vi "CRYO_MASTER_FULL_IP.vi"() -> ()   [LabVIEW 2017] (continued)
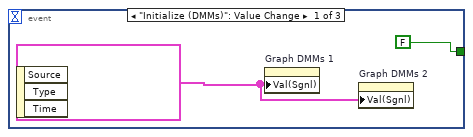
[diagram p2: hidden frame]
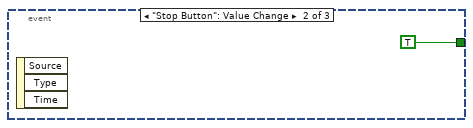
[diagram p3: hidden frame]
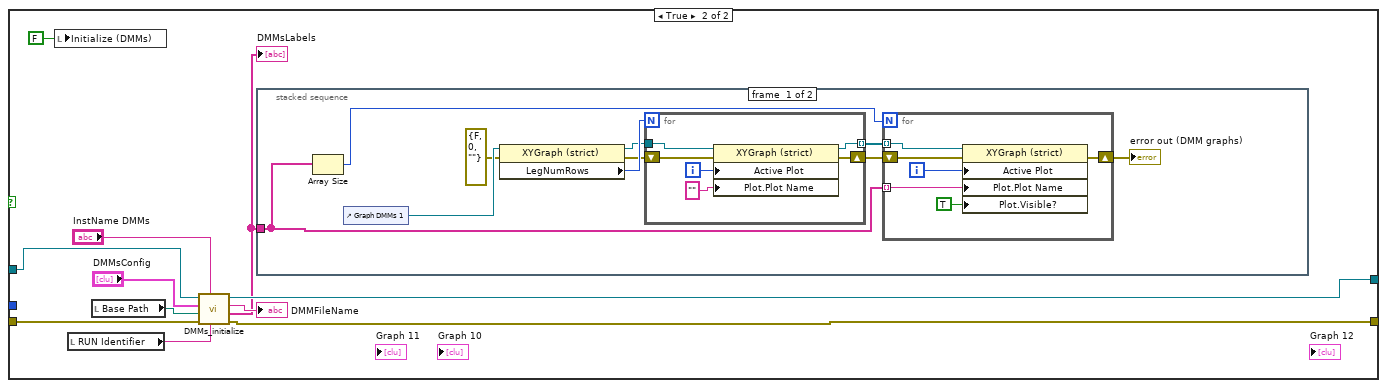
[diagram p5: hidden frame]
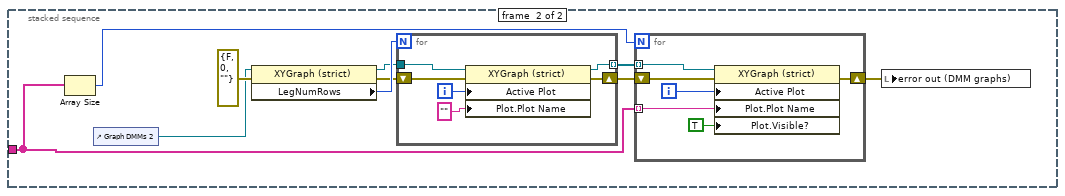
[diagram p6: hidden frame]
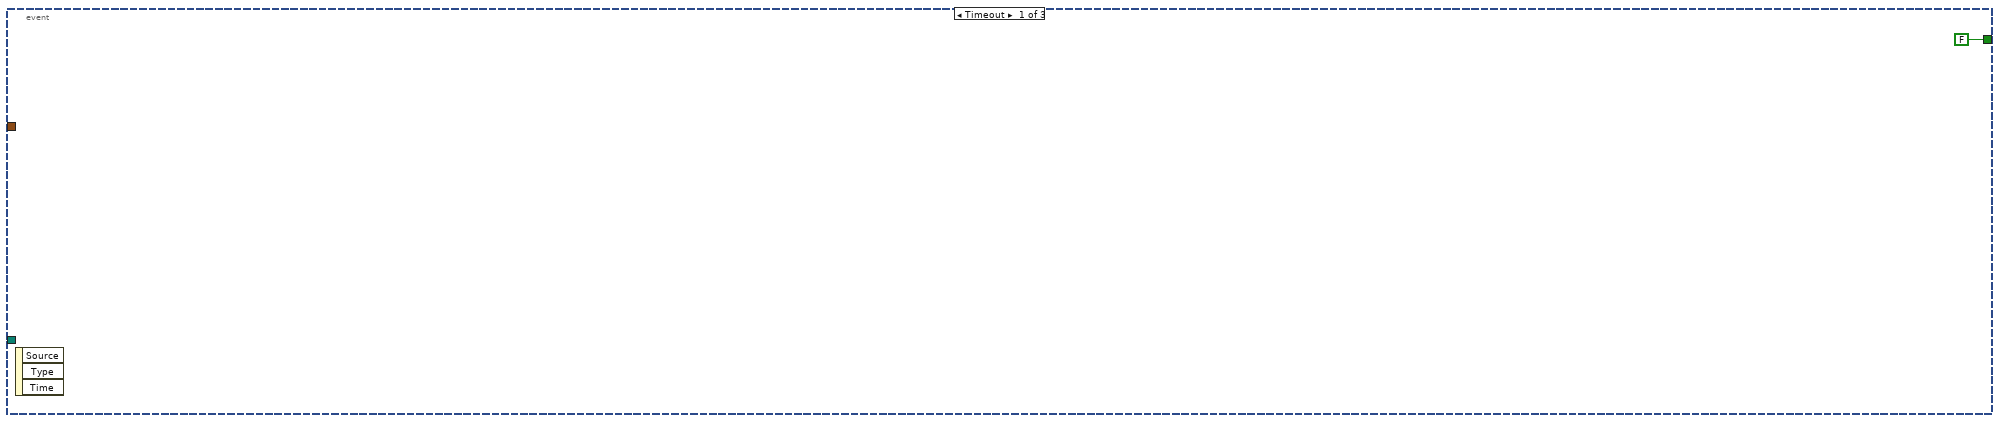
[diagram p7: hidden frame]
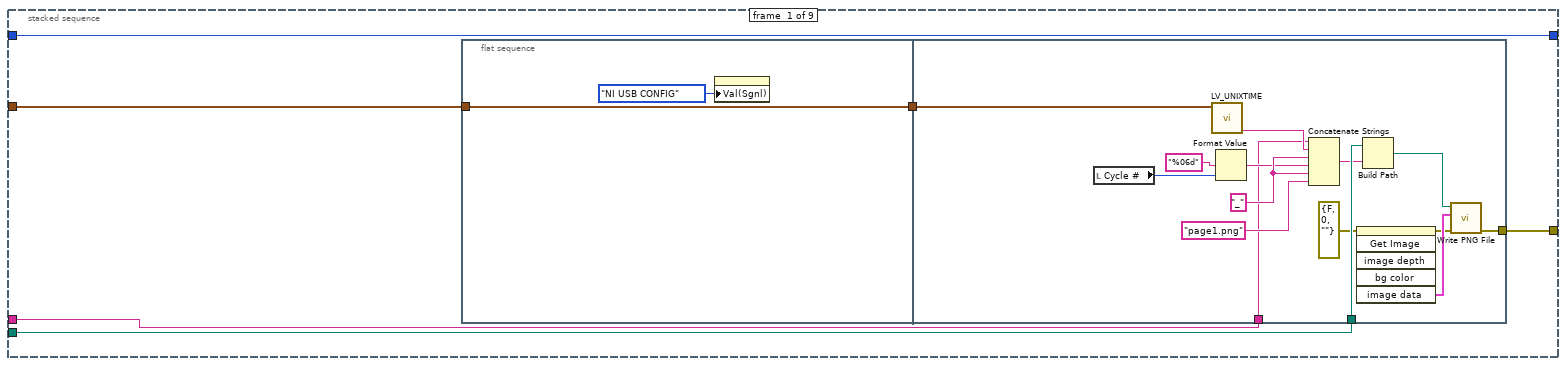
[diagram p8: hidden frame]
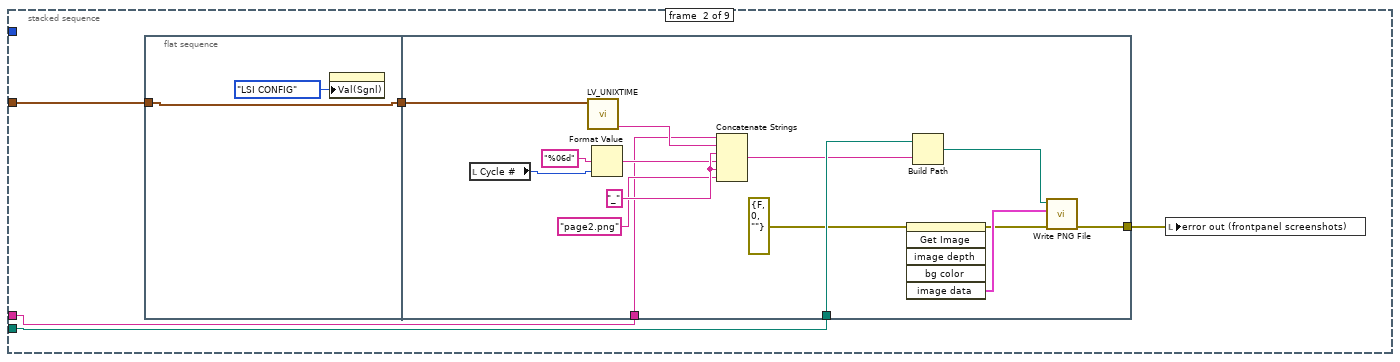
[diagram p9: hidden frame]
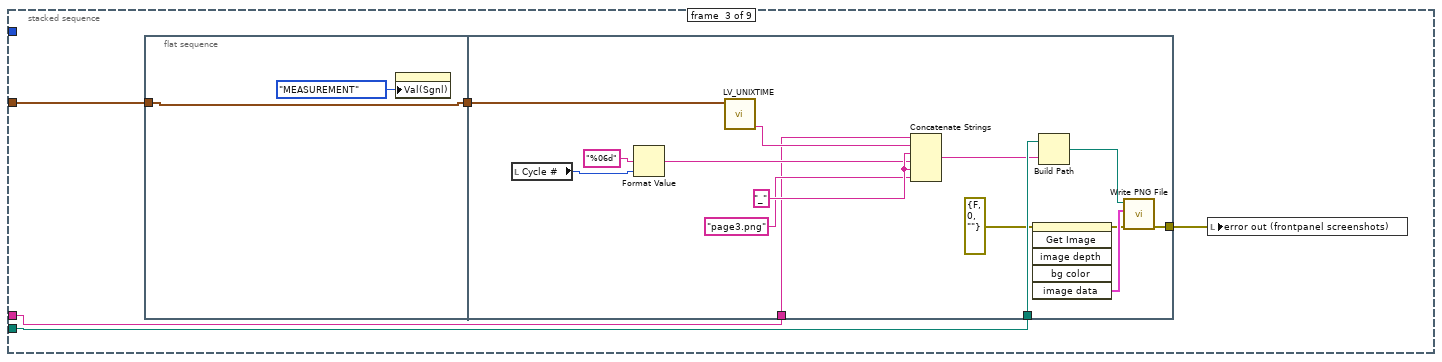
[diagram p10: hidden frame]
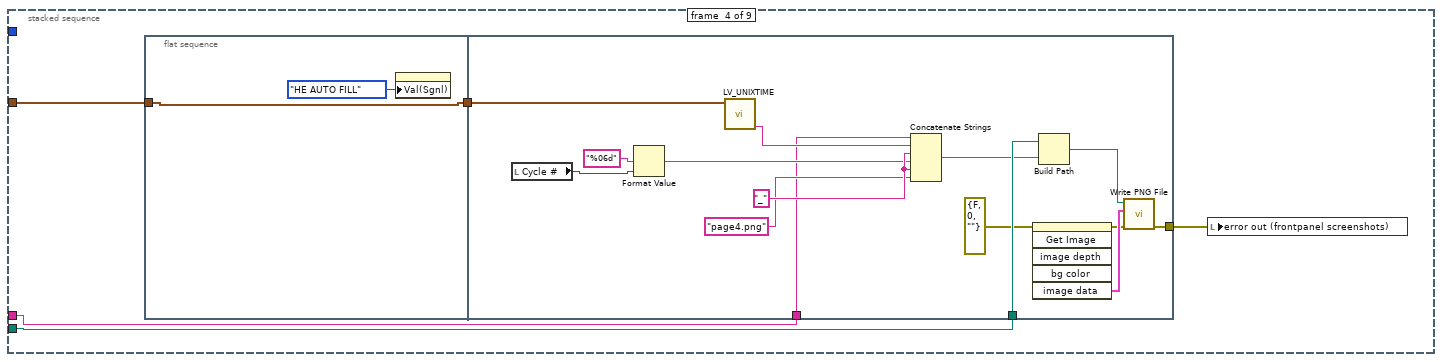
[diagram p11: hidden frame]
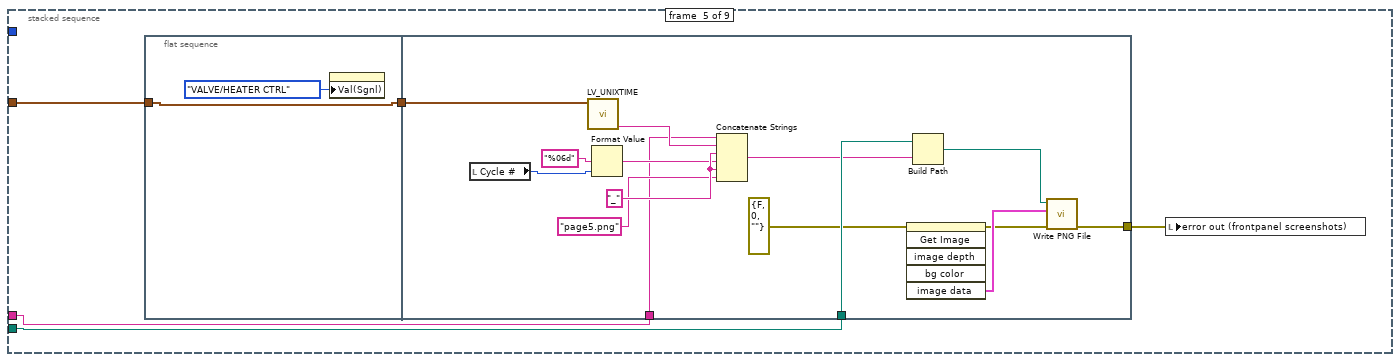
[diagram p12: hidden frame]
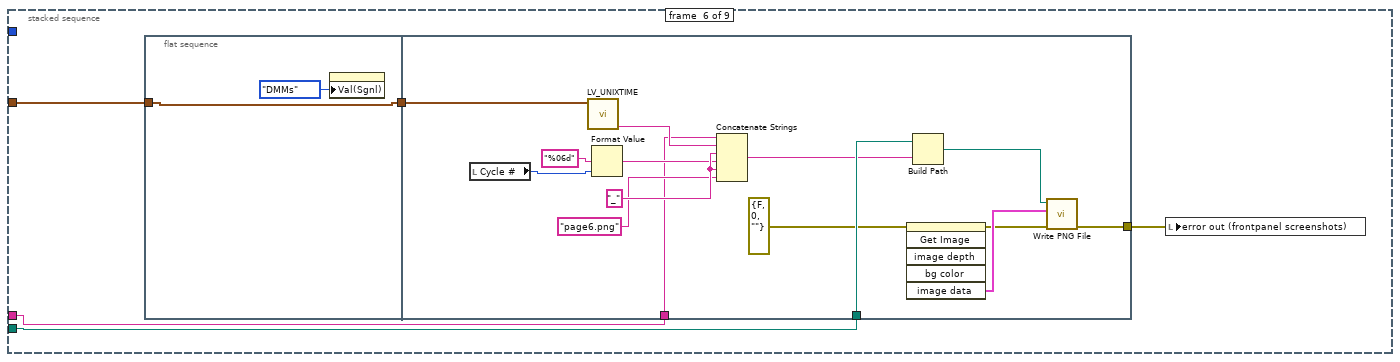
[diagram p13: hidden frame]
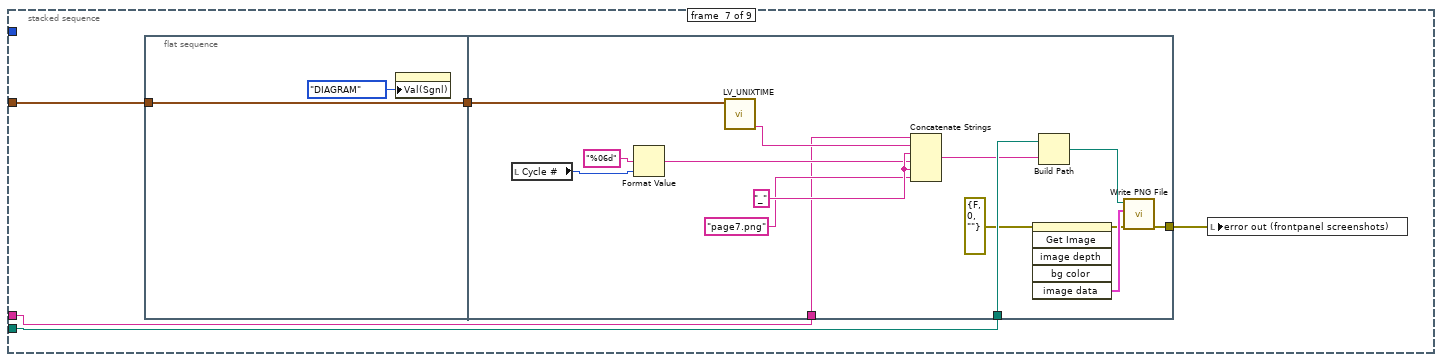
[diagram p14: hidden frame]
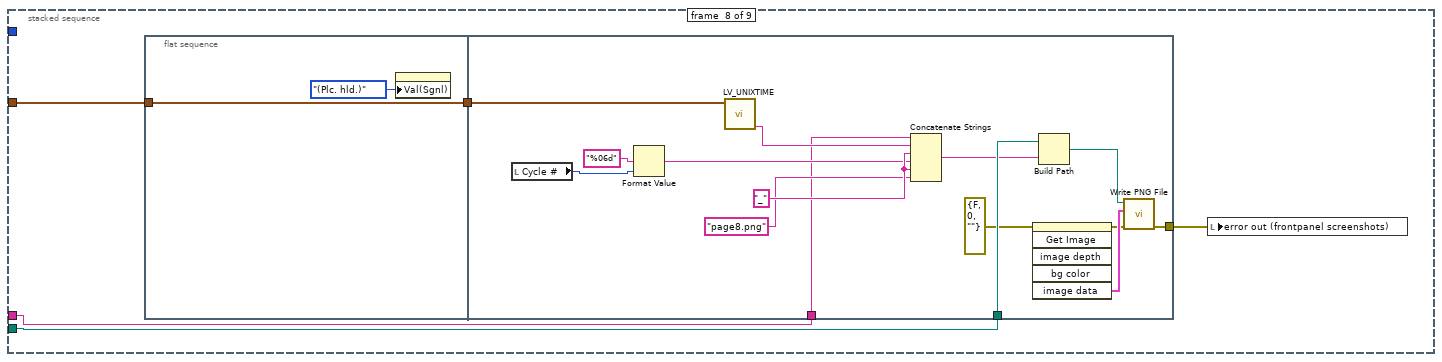
[diagram p15: hidden frame]
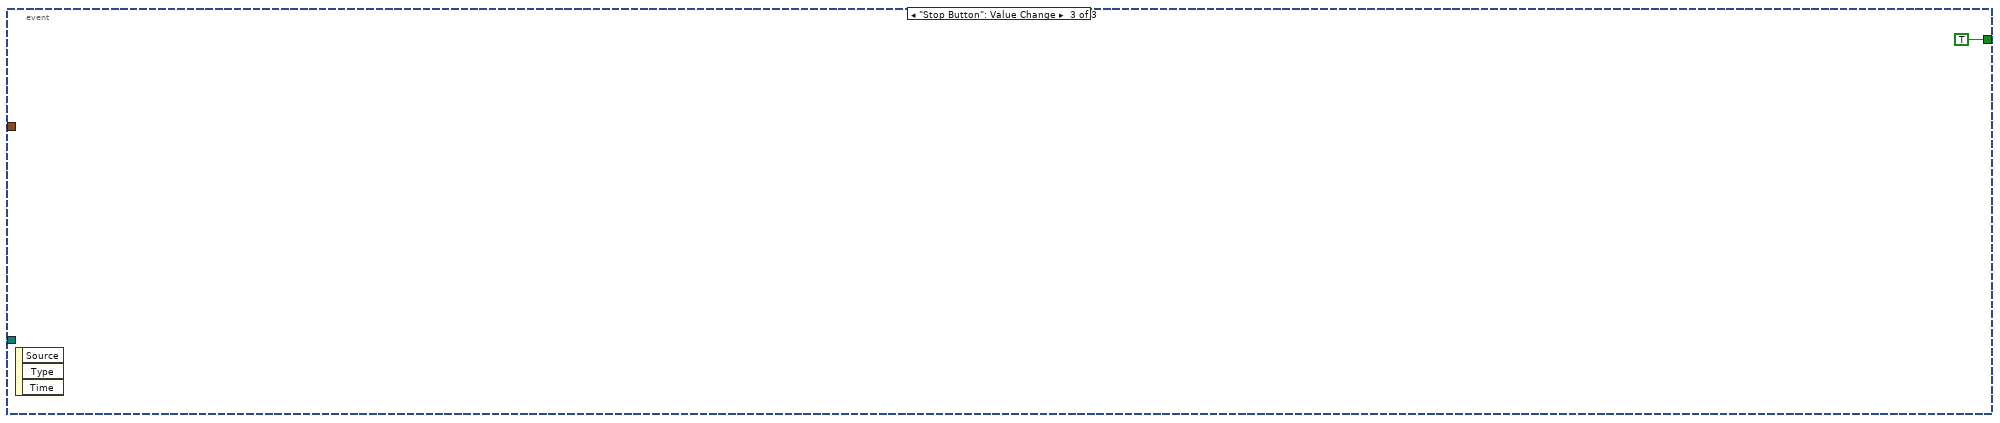
[diagram p16: hidden frame]
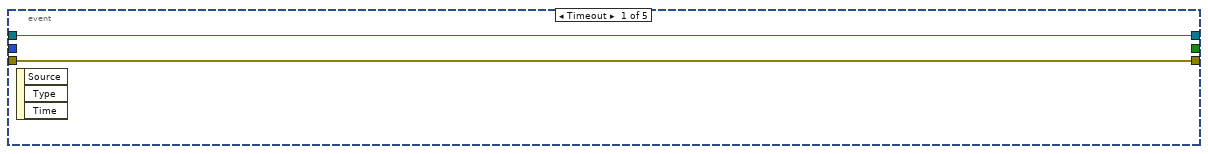
[diagram p18: hidden frame]
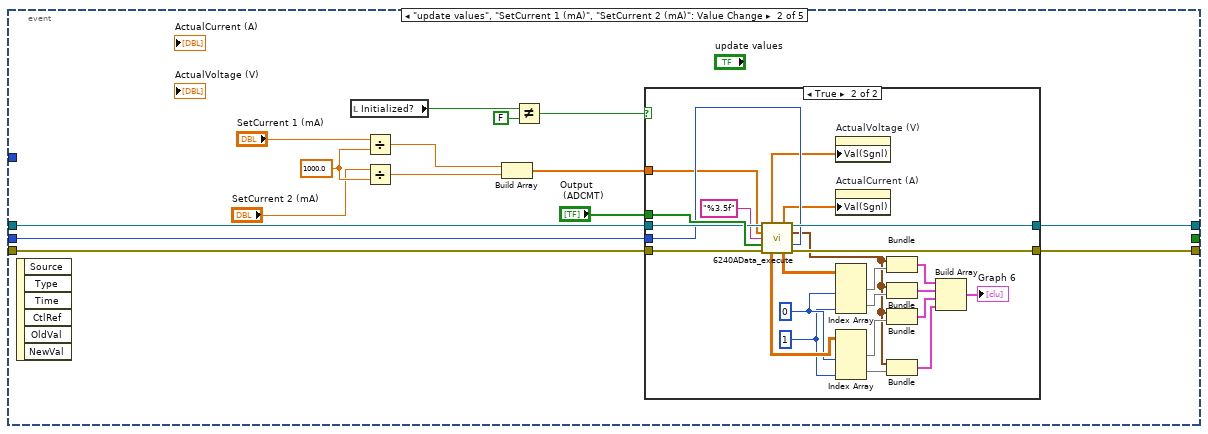
[diagram p19: hidden frame]
                  frame #0 {
                    n725 = flat-sequence {
                      tunnel: w1528 -> [w1530]
                      tunnel: w1527 -> [w1529]
                      tunnel: w1527 -> [w1598]
                      frame #0 {
                        n726 = stacked-sequence {
                          tunnel: w1530 -> [w1537 w1541 _ _ _ _]
                          tunnel: w1529 -> [_ _ w1555 w1564 w1573 w1582]
                          frame #0 {
                            n727 = local read "L_low (%)"() -> (w1536:dbl)
                            n728 = local read "Fill state"() -> (w1534:bool)
                            n729 = Less?(x=w1537, y=w1536) -> (x < y?=w1533:bool)
                            n730 = Equal?(x=w1534, y=FALSE) -> (x = y?=w1532:bool)
                            n731 = And(x=w1533, y=w1532) -> (x .and. y?=w1531:bool)
                            n732 = case shown="False" w1531 {
                              frame False {
                              }
                              frame True {
                                w1539 = TRUE ("Value (Signaling)")
                                n733 = property on="Fill state" class="Bool (strict)"("Val(Sgnl)"=w1539) -> ()  [unwired: 2 in, 2 out]
                                n734 = Not(x=w1539) -> (.not. x?=w1538:bool)
                                n735 = property on="Fill (false)" class="Bool (strict)"("Val(Sgnl)"=w1538) -> ()  [unwired: 2 in, 2 out]
                              }
                            }
                          }
                          frame #1 {
                            n736 = local read "L_high (%)"() -> (w1542:dbl)
                            n737 = local read "Fill state"() -> (w1545:bool)
                            n738 = Greater?(x=w1541, y=w1542) -> (0:w1540:bool)
                            n739 = Equal?(x=w1545, y=TRUE) -> (x = y?=w1544:bool)
                            n740 = And(x=w1540, y=w1544) -> (x .and. y?=w1543:bool)
                            n741 = case shown="True" w1543 {
                              frame False {
                              }
                              frame True {
                                w1547 = FALSE ("Value (Signaling)")
                                n742 = property on="Fill state" class="Bool (strict)"("Val(Sgnl)"=w1547) -> ()  [unwired: 2 in, 2 out]
                                n743 = Not(x=w1547) -> (.not. x?=w1548:bool)
                                n744 = property on="Fill (false)" class="Bool (strict)"("Val(Sgnl)"=w1548) -> ()  [unwired: 2 in, 2 out]
                              }
                            }
                          }
                          frame #2 {
                            n745 = local read "P_1_low (Pa)"() -> (w1554:dbl)
                            n746 = property on="state 1" class="Bool (strict)"() -> ("Value"=w1552:bool)  [unwired: 2 in, 2 out]
                            n747 = Less?(x=w1555, y=w1554) -> (x < y?=w1551:bool)
                            n748 = Equal?(x=w1552, y=FALSE) -> (x = y?=w1550:bool)
                            n749 = And(x=w1550, y=w1551) -> (x .and. y?=w1549:bool)
                            n750 = case shown="True" w1549 {
                              frame False {
                              }
                              frame True {
                                w1557 = TRUE ("Value (Signaling)")
                                n751 = property on="state 1" class="Bool (strict)"("Val(Sgnl)"=w1557) -> ()  [unwired: 2 in, 2 out]
                                n752 = Not(x=w1557) -> (.not. x?=w1556:bool)
                                n753 = property on="state 1 (false)" class="Bool (strict)"("Val(Sgnl)"=w1556) -> ()  [unwired: 2 in, 2 out]
                              }
                            }
                          }
                          frame #3 {
                            n754 = local read "P_1_high (Pa)"() -> (w1563:dbl)
                            n755 = property on="state 1" class="Bool (strict)"() -> ("Value"=w1561:bool)  [unwired: 2 in, 2 out]
                            n756 = Greater?(x=w1564, y=w1563) -> (0:w1560:bool)
                            n757 = Equal?(x=w1561, y=TRUE) -> (x = y?=w1559:bool)
                            n758 = And(x=w1559, y=w1560) -> (x .and. y?=w1558:bool)
                            n759 = case shown="True" w1558 {
                              frame False {
                              }
                              frame True {
                                w1566 = FALSE ("Value (Signaling)")
                                n760 = property on="state 1" class="Bool (strict)"("Val(Sgnl)"=w1566) -> ()  [unwired: 2 in, 2 out]
                                n761 = Not(x=w1566) -> (.not. x?=w1565:bool)
                                n762 = property on="state 1 (false)" class="Bool (strict)"("Val(Sgnl)"=w1565) -> ()  [unwired: 2 in, 2 out]
                              }
                            }
                          }
                          frame #4 {
                            n763 = local read "P_2_low (Pa)"() -> (w1572:dbl)
                            n764 = property on="state 2" class="Bool (strict)"() -> ("Value"=w1567:bool)  [unwired: 2 in, 2 out]
                            n765 = Less?(x=w1573, y=w1572) -> (x < y?=w1570:bool)
                            n766 = Equal?(x=w1567, y=FALSE) -> (x = y?=w1569:bool)
                            n767 = And(x=w1569, y=w1570) -> (x .and. y?=w1568:bool)
                            n768 = case shown="True" w1568 {
                              frame False {
                              }
                              frame True {
                                w1574 = TRUE ("Value (Signaling)")
                                n769 = property on="state 2" class="Bool (strict)"("Val(Sgnl)"=w1574) -> ()  [unwired: 2 in, 2 out]
                                n770 = Not(x=w1574) -> (.not. x?=w1575:bool)
                                n771 = property on="state 2 (false)" class="Bool (strict)"("Val(Sgnl)"=w1575) -> ()  [unwired: 2 in, 2 out]
                              }
                            }
                          }
                          frame #5 {
                            n772 = local read "P_2_high (Pa)"() -> (w1581:dbl)
                            n773 = property on="state 2" class="Bool (strict)"() -> ("Value"=w1576:bool)  [unwired: 2 in, 2 out]
                            n774 = Greater?(x=w1582, y=w1581) -> (0:w1579:bool)
                            n775 = Equal?(x=w1576, y=TRUE) -> (x = y?=w1578:bool)
                            n776 = And(x=w1578, y=w1579) -> (x .and. y?=w1577:bool)
                            n777 = case shown="True" w1577 {
                              frame False {
                              }
                              frame True {
                                w1583 = FALSE ("Value (Signaling)")
                                n778 = property on="state 2" class="Bool (strict)"("Val(Sgnl)"=w1583) -> ()  [unwired: 2 in, 2 out]
                                n779 = Not(x=w1583) -> (.not. x?=w1584:bool)
                                n780 = property on="state 2 (false)" class="Bool (strict)"("Val(Sgnl)"=w1584) -> ()  [unwired: 2 in, 2 out]
                              }
                            }
                          }
                        }
                      }
                      frame #1 {
                        n781 = property on="Fill state" class="Bool (strict)"() -> ("Value"=w1585:bool)  [unwired: 2 in, 2 out]
                        n782 = case shown="True" w1585 {
                          frame False {
                            n783 = property on="V1 (N.O.)" class="Bool (strict)"("Val(Sgnl)"=TRUE ("V1 (N.O.)")) -> ()  [unwired: 2 in, 2 out]
                            n784 = property on="V2 (N.C.)" class="Bool (strict)"("Val(Sgnl)"=FALSE ("Value (Signaling)")) -> ()  [unwired: 2 in, 2 out]
                          }
                          frame True {
                            n785 = property on="state 1" class="Bool (strict)"() -> ("Value"=w1589:bool)  [unwired: 2 in, 2 out]
                            n786 = property on="state 2" class="Bool (strict)"() -> ("Value"=w1588:bool)  [unwired: 2 in, 2 out]
                            n787 = case shown="True" w1589 {
                              frame False {
                                n788 = property on="V1 (N.O.)" class="Bool (strict)"("Val(Sgnl)"=TRUE ("Value (Signaling)")) -> ()  [unwired: 2 in, 2 out]
                                n789 = local write "Status V1 CTRL"(enum16{"Pressurize", "Release"}."Release" ("Status V1 CTRL")) -> ()
                              }
                              frame True {
                                n790 = property on="V1 (N.O.)" class="Bool (strict)"("Val(Sgnl)"=FALSE ("V1 (N.O.)")) -> ()  [unwired: 2 in, 2 out]
                                n791 = local write "Status V1 CTRL"(enum16{"Pressurize", "Release"}."Pressurize" ("Status V1 CTRL")) -> ()
                              }
                            }
                            n792 = case shown="True" w1588 {
                              frame False {
                                n793 = property on="V2 (N.C.)" class="Bool (strict)"("Val(Sgnl)"=FALSE ("Value (Signaling)")) -> ()  [unwired: 2 in, 2 out]
                                n794 = local write "Status V2 CTRL"(enum16{"Pressurize", "Release"}."Release" ("Status V2 CTRL")) -> ()
                              }
                              frame True {
                                n795 = property on="V2 (N.C.)" class="Bool (strict)"("Val(Sgnl)"=TRUE ("Value (Signaling)")) -> ()  [unwired: 2 in, 2 out]
                                n796 = local write "Status V2 CTRL"(enum16{"Pressurize", "Release"}."Pressurize" ("Status V2 CTRL")) -> ()
                              }
                            }
                          }
                        }
                      }
                      frame #2 {
                        n797 = Greater?(x=w1598, y="P_safelimit_high (Pa)") -> (0:w1600:bool)
                        n798 = Less?(x=w1598, y="P_safelimit_low (Pa)") -> (x < y?=w1602:bool)
                        n799 = Or(x=w1600, y=w1602) -> (x .or. y?=w1603:bool)
                        n800 = case shown="False" w1603 {
                          frame False {
                          }
                          frame True {
                            w1604 = FALSE ("Value (Signaling)")
                            w1606 = FALSE ("Value (Signaling)")
                            n801 = property on="V2 (N.C.)" class="Bool (strict)"("Val(Sgnl)"=FALSE ("V1 (N.O.)")) -> ()  [unwired: 2 in, 2 out]
                            n802 = property on="state 1" class="Bool (strict)"("Val(Sgnl)"=w1604) -> ()  [unwired: 2 in, 2 out]
                            n803 = property on="V1 (N.O.)" class="Bool (strict)"("Val(Sgnl)"=TRUE ("V1 (N.O.)")) -> ()  [unwired: 2 in, 2 out]
                            n804 = property on="state 2" class="Bool (strict)"("Val(Sgnl)"=w1606) -> ()  [unwired: 2 in, 2 out]
                            n805 = Not(x=w1604) -> (.not. x?=w1605:bool)
                            n806 = Not(x=w1606) -> (.not. x?=w1607:bool)
                            n807 = property on="state 1 (false)" class="Bool (strict)"("Val(Sgnl)"=w1605) -> ()  [unwired: 2 in, 2 out]
                            n808 = property on="state 2 (false)" class="Bool (strict)"("Val(Sgnl)"=w1607) -> ()  [unwired: 2 in, 2 out]
                          }
                        }
                      }
                    }
                  }
                  frame #1 {
                    n809 = property on="V2 (N.C.)" class="Bool (strict)"() -> ("Value"=w1617:bool)  [unwired: 2 in, 2 out]
                    n810 = property on="V1 (N.O.)" class="Bool (strict)"() -> ("Value"=w1628:bool)  [unwired: 2 in, 2 out]
                    n811 = local read "P_1_high (Pa)"() -> (w1622:dbl)
                    n812 = local read "P_2_high (Pa)"() -> (w1620:dbl)
                    n813 = local read "P_1_low (Pa)"() -> (w1623:dbl)
                    n814 = local read "P_2_low (Pa)"() -> (w1621:dbl)
                    n815 = local read "L_high (%)"() -> (w1618:dbl)
                    n816 = local read "L_low (%)"() -> (w1619:dbl)
                    n817 = local read "Pav (Pa)"() -> (w1611:dbl)
                    n818 = local read "Lav (%)"() -> (w1610:dbl)
                    n819 = Boolean To (0,1)(Boolean=w1617) -> (0, 1=w1616:i16)
                    n820 = Boolean To (0,1)(Boolean=w1628) -> (0, 1=w1629:i16)
                    n821 = local read "File Refn DewarCTRL"() -> (w1624:refnum<file>)
                    n822 = local read "Cycle #"() -> (w1627:u32)
                    n823 = Build Array(w1611, w1610, w1623, w1622, w1621, w1620, w1619, w1618, w1629, w1616) -> (w1615:dbl[])
                    n824 = Get Date/Time In Seconds() -> (seconds since 1Jan1904=w1625:timestamp)
                    n825 = call "FileWrite.vi"("DataArray"=w1615, "Time Stamp"=w1625, "Error In"=errorcluster {"status"=FALSE, "code"=0, "source"=""}, "FileFormat"=string[] ["%4.5e", "%4.2f", "%4.4e", "%4.4e", "%4.4e", "%4.4e", "%4.4e", "%d", "%d"] ("Array"), "Index"=w1627, "refnum in"=w1624) -> ("Error Out"=→"Error Out (Dewar CTRL":errorcluster, "Byte Stream File Refnum"=w1614:refnum<file>)  [unwired: 4 in]
                    n826 = local write "File Refn DewarCTRL"(w1614) -> ()
                  }
                }
              }
            }
          }
          frame True {
            w1668 = "_"
            w1637 = FALSE ("auto cleanup")
            w1673 = 1 items=["one channel for each line", "one channel for all lines"] ("line grouping")
            n827 = flat-sequence {
              frame #0 {
                w1688 = FALSE ("V1 (N.O.)")
                n828 = local write "V2 (N.C.)"(FALSE ("V1 (N.O.)")) -> ()
                n829 = local write "V1 (N.O.)"(TRUE ("V1 (N.O.)")) -> ()
                n830 = local write "state 2"(w1688) -> ()
                n831 = local write "state 1"(w1688) -> ()
                n832 = local write "Fill state"(w1688) -> ()
                n833 = Not(x=w1688) -> (.not. x?=w1690:bool)
                n834 = Not(x=w1688) -> (.not. x?=w1689:bool)
                n835 = local write "state 1 (false)"(w1689) -> ()
                n836 = local write "state 2 (false)"(w1689) -> ()
                n837 = local write "Fill (false)"(w1690) -> ()
              }
            }
            n838 = Get Date/Time In Seconds() -> (seconds since 1Jan1904=w1685:timestamp)
            n839 = call "LV_UNIXTIME.vi"("current time"=w1685) -> ("date/time string"=w1663:string)  [unwired: 9 in, 1 out]
            n840 = Concatenate Strings(w1663, "_DO" ("new task name")) -> (w1682:string)
            n841 = Concatenate Strings(w1662, w1668, w1663, w1668) -> (w1644:string)
            n842 = Concatenate Strings(w1644, "DEWAR.csv" ("string")) -> (w1643:string)
            n843 = Concatenate Strings(w1644, "USB_DOUT.csv" ("string")) -> (w1647:string)
            n844 = Build Path(base path=w1645, name or relative path=w1643) -> (appended path=w1642:path)
            n845 = Build Path(base path=w1645, name or relative path=w1647) -> (appended path=w1667:path)
            n846 = Open/Create/Replace File(file path (use dialog)=w1667, error in=w1653, operation (0:open)=T19."open or create") -> (refnum out=w1665:refnum<file>, error out=w1652:errorcluster)  [unwired: 3 in, 1 out]
            n847 = call "FileIntialize.vi"("Error In"=w1652, "Labels"="DOUT Labels", "refnum in"=w1665) -> ("Error Out"=w1639:errorcluster, "File Refnum"=→"File Refn USB DO":refnum<file>)  [unwired: 7 in]
            n848 = Open/Create/Replace File(file path (use dialog)=w1642, error in=w1639, operation (0:open)=T19."open or create") -> (refnum out=w1650:refnum<file>, error out=w1651:errorcluster)  [unwired: 3 in, 1 out]
            n849 = call "FileIntialize.vi"("Error In"=w1651, "Labels"=string[] ["P_av", "L_av", "P_1_low", "P_1_high", "P_2_low", "P_2_high", "L_low", "L_high", "V1(NO)", "V2(NC)"], "refnum in"=w1650) -> ("Error Out"=w1638:errorcluster, "File Refnum"=→"File Refn DewarCTRL":refnum<file>)  [unwired: 7 in]
            n850 = Index Array(array="DOUT Physical CH", index=2) -> (element=w1655:tag)
            n851 = Index Array(array="DOUT Physical CH", index=1) -> (element=w1658:tag)
            n852 = Index Array(array="DOUT Physical CH", index=0) -> (element=w1660:tag)
            n853 = call <vilib>:"DAQmx Create Task.vi"("new task name"=w1682, "auto cleanup"=FALSE, "error in"=w1638) -> ("task out"=w1683:refnum<k21>, "error out"=w1684:errorcluster)  [unwired: 11 in]
            n854 = call-poly <vilib>:"DAQmx Create Virtual Channel.vi"("task in"=w1683, "lines"=w1660, "line grouping"=w1673, "error in"=w1684) -> ("task out"=w1686:refnum<k21>, "error out"=w1687:errorcluster)  [unwired: 10 in]
            n855 = call-poly <vilib>:"DAQmx Create Virtual Channel.vi"("task in"=w1686, "lines"=w1658, "line grouping"=w1673, "error in"=w1687) -> ("task out"=w1672:refnum<k21>, "error out"=w1670:errorcluster)  [unwired: 10 in]
            n856 = call-poly <vilib>:"DAQmx Create Virtual Channel.vi"("task in"=w1672, "lines"=w1655, "line grouping"=w1673, "error in"=w1670) -> ("task out"=w1671:refnum<k21>, "error out"=w1669:errorcluster)  [unwired: 10 in]
            n857 = call <vilib>:"DAQmx Start Task.vi"("task/channels in"=w1671, "error in"=w1669) -> ("task out"=w1677:refnum<k21>, "error out"=w1675:errorcluster)  [unwired: 12 in]
            n858 = Build Array(w1637, w1637, w1637) -> (w1678:bool[])
            n859 = call <vilib>:"DAQmx Write (Digital 1D Bool NChan 1Samp 1Line).vi"("task/channels in"=w1677, "data"=w1678, "timeout"=10.0, "error in"=w1675) -> ("task out"=→"DOUT task out":refnum<k21>, "error out"=w1674:errorcluster)  [unwired: 9 in, 1 out]
          }
        }
      }
    }
    "error out (USB6210/6218 DOUT)" <- w806
    n860 = flat-sequence {
      tunnel: w801 -> [w1274]
      tunnel: [w1269] -> w800
      tunnel: [w1267] -> w799
      tunnel: [w1266] -> w798
      tunnel: [w1265] -> w797
      tunnel: w802 -> [w1261]
      frame #0 {
        w1268 = T20 [] ("appended array")
        n861 = Unbundle By Name(w1261) -> ("TimeArray"=w1257:timestamp[], "DataArrayConv"=w1272:dbl[][], "LDArray"=w1271:dbl[])
        "TimeArray (USB6218)" <- w1257
        n862 = Unbundle By Name(w1274) -> ("ReadLeakDet?"=w1273:bool, "LabelLD"=w1276:string, "Labels"=w1270:string[])  [unwired: 1 out]
        n863 = case shown="True" w1273 {
          tunnel: w1276 -> [_ w1284]
          tunnel: w1272 -> [w1278 w1283]
          tunnel: w1271 -> [_ w1282]
          tunnel: [w1278 w1281] -> w1259
          tunnel: w1270 -> [w1277 w1280]
          tunnel: [w1277 w1279] -> w1262
          frame False {
          }
          frame True {
            n864 = Build Array (concatenate)(w1283, w1282) -> (w1281:dbl[][])
            n865 = Build Array (concatenate)(w1280, w1284) -> (w1279:string[])
          }
        }
        "All Labels (USB6218)" <- w1262
        "DataArrayConv (USB6218)" <- w1259
        n866 = Array Size(array=w1257) -> (size(s)=→"TimeArray size (6218)":i32)
        n867 = local read "Plot selecter (USB6218)\n    1      2     3     4"() -> (w1264:bool[][])
        n868 = control-ref of="Plot selecter (USB6218)\n    1      2     3     4"() -> (w1260:refnum<vi>)
        n869 = Array Size(array=w1262) -> (size(s)=w1263:i32)
        n870 = Array Size(array=w1262) -> (size(s)=w1275:i32)
        n871 = Array Size(array=w1259) -> (size(s)=→"DataArraySize (6218)":i32[])
        n872 = property on="Property Node" class="Arr (strict)"(reference=w1260, "Number of Rows"=w1263) -> ()  [unwired: 1 in, 2 out]
        n873 = for {
          N: w1275 -> [_]
          tunnel: w1259 -> [w1305]
          tunnel: w1257 -> [w1306]
          shift-right: [w1300] -> w1267
          shift-left: w1268 -> [w1303]
          shift-right: [w1298] -> w1265
          shift-left: w1268 -> [w1301]
          shift-right: [w1299] -> w1269
          shift-left: w1268 -> [w1297]
          shift-right: [w1296] -> w1266
          shift-left: w1268 -> [w1295]
          tunnel: w1264 -> [w1294]
          i -> [w1289]
          n874 = Index Array(array=w1305, index (col)=w1289) -> (element=w1304:dbl[])  [unwired: 1 in]
          n875 = Index Array(array=w1294, index (row) #1=w1289, index (col) #1=0 ("index (row)"), index (row) #2=w1289, index (col) #2=1 ("index (row)"), index (row) #3=w1289, index (col) #3=2 ("index (row)"), index (row) #4=w1289, index (col) #4=3 ("index (row)")) -> (element #1=w1288:bool, element #2=w1287:bool, element #3=w1286:bool, element #4=w1285:bool)
          n876 = Bundle("TimeArray"=w1306, "DataArrayConv"=w1304) -> (w1302:T23)  [unwired: 1 in]
          n877 = stacked-sequence {
            tunnel: w1288 -> [w1310 _ _ _]
            tunnel: w1303 -> [_ w1318 _ _]
            tunnel: w1286 -> [_ _ w1326 _]
            tunnel: w1302 -> [w1307 w1316 w1325 w1331]
            tunnel: w1285 -> [_ _ _ w1334]
            tunnel: w1301 -> [_ _ _ w1333]
            tunnel: [_ _ _ w1332] -> w1298
            tunnel: [_ w1317 _ _] -> w1300
            tunnel: [w1309 _ _ _] -> w1299
            tunnel: w1297 -> [w1308 _ _ _]
            tunnel: [_ _ w1324 _] -> w1296
            tunnel: w1295 -> [_ _ w1323 _]
            tunnel: w1287 -> [_ w1315 _ _]
            frame #0 {
              n878 = case shown="True" w1310 {
                tunnel: [w1311 w1314] -> w1309
                tunnel: w1307 -> [_ w1313]
                tunnel: w1308 -> [w1311 w1312]
                frame False {
                }
                frame True {
                  n879 = Build Array (concatenate)(w1312, w1313) -> (w1314:T20)
                }
              }
            }
            frame #1 {
              n880 = case shown="True" w1315 {
                tunnel: w1318 -> [w1319 w1322]
                tunnel: [w1319 w1321] -> w1317
                tunnel: w1316 -> [_ w1320]
                frame False {
                }
                frame True {
                  n881 = Build Array (concatenate)(w1322, w1320) -> (w1321:T20)
                }
              }
            }
            frame #2 {
              n882 = case shown="True" w1326 {
                tunnel: [w1327 w1330] -> w1324
                tunnel: w1325 -> [_ w1329]
                tunnel: w1323 -> [w1327 w1328]
                frame False {
                }
                frame True {
                  n883 = Build Array (concatenate)(w1328, w1329) -> (w1330:T20)
                }
              }
            }
            frame #3 {
              n884 = case shown="True" w1334 {
                tunnel: [w1335 w1338] -> w1332
                tunnel: w1331 -> [_ w1337]
                tunnel: w1333 -> [w1335 w1336]
                frame False {
                }
                frame True {
                  n885 = Build Array (concatenate)(w1336, w1337) -> (w1338:T20)
                }
              }
            }
          }
        }
      }
    }
    n886 = Build Array (concatenate)(w770, w771) -> (w768:dbl[])
    n887 = Build Array (concatenate)(w773, w772) -> (w769:string[])
    n888 = local read "Plot selecter LSI218(2)\n    1      2     3     4"() -> (w828:bool[][])
    n889 = local read "Plot selecter LSI218(1)\n    1      2     3     4"() -> (w829:bool[][])
    n890 = for {
      N: 48 -> [_]
      tunnel: w844 -> [w1792]
      tunnel: w843 -> [w1789]
      tunnel: w829 -> [w1773]
      tunnel: w828 -> [w1774]
      shift-right: [w1790] -> w842
      shift-left: w840 -> [w1791]
      shift-right: [w1785] -> w837
      shift-left: w840 -> [w1786]
      shift-right: [w1784] -> w835
      shift-left: w840 -> [w1783]
      shift-right: [w1782] -> w833
      shift-left: w840 -> [w1781]
      i -> [w1779]
      n891 = Index Array(array=w1789, index (col)=w1779) -> (element=w1788:dbl[])  [unwired: 1 in]
      n892 = Less?(x=w1779, y=24) -> (x < y?=w1780:bool)
      n893 = case shown="True" w1780 {
        tunnel: [w1797 w1815] -> w1778
        tunnel: [w1796 w1814] -> w1777
        tunnel: [w1795 w1812] -> w1776
        tunnel: [w1794 w1811] -> w1775
        tunnel: w1773 -> [_ w1810]
        tunnel: w1774 -> [w1804 _]
        tunnel: w1779 -> [w1799 w1807]
        frame False {
          n894 = Subtract(x=w1799, y=24) -> (x-y=w1803:i32)
          n895 = Index Array(array=w1804, index (row) #1=w1803, index (col) #1=0 ("index (row)"), index (row) #2=w1803, index (col) #2=1 ("index (row)"), index (row) #3=w1803, index (col) #3=2 ("index (row)"), index (row) #4=w1803, index (col) #4=3 ("index (row)")) -> (element #1=w1797:bool, element #2=w1796:bool, element #3=w1795:bool, element #4=w1794:bool)
        }
        frame True {
          n896 = Index Array(array=w1810, index (row) #1=w1807, index (col) #1=0 ("index (row)"), index (row) #2=w1807, index (col) #2=1 ("index (row)"), index (row) #3=w1807, index (col) #3=2 ("index (row)"), index (row) #4=w1807, index (col) #4=3 ("index (row)")) -> (element #1=w1815:bool, element #2=w1814:bool, element #3=w1812:bool, element #4=w1811:bool)
        }
      }
      n897 = Bundle("TimeArray"=w1792, "DataArray"=w1788) -> (w1787:T26)  [unwired: 1 in]
      n898 = stacked-sequence {
        tunnel: w1791 -> [w1819 _ _ _]
        tunnel: [w1818 _ _ _] -> w1790
        tunnel: w1787 -> [w1817 w1827 w1835 w1843]
        tunnel: w1786 -> [_ w1826 _ _]
        tunnel: [_ w1825 _ _] -> w1785
        tunnel: [_ _ w1834 _] -> w1784
        tunnel: w1783 -> [_ _ w1833 _]
        tunnel: [_ _ _ w1842] -> w1782
        tunnel: w1781 -> [_ _ _ w1841]
        tunnel: w1778 -> [w1816 _ _ _]
        tunnel: w1777 -> [_ w1824 _ _]
        tunnel: w1776 -> [_ _ w1832 _]
        tunnel: w1775 -> [_ _ _ w1840]
        frame #0 {
          n899 = case shown="False" w1816 {
            tunnel: w1817 -> [_ w1821]
            tunnel: w1819 -> [w1820 w1823]
            tunnel: [w1820 w1822] -> w1818
            frame False {
            }
            frame True {
              n900 = Build Array (concatenate)(w1823, w1821) -> (w1822:T1)
            }
          }
        }
        frame #1 {
          n901 = case shown="True" w1824 {
            tunnel: [w1828 w1831] -> w1825
            tunnel: w1827 -> [_ w1830]
            tunnel: w1826 -> [w1828 w1829]
            frame False {
            }
            frame True {
              n902 = Build Array (concatenate)(w1829, w1830) -> (w1831:T1)
            }
          }
        }
        frame #2 {
          n903 = case shown="True" w1832 {
            tunnel: [w1836 w1839] -> w1834
            tunnel: w1835 -> [_ w1838]
            tunnel: w1833 -> [w1836 w1837]
            frame False {
            }
            frame True {
              n904 = Build Array (concatenate)(w1837, w1838) -> (w1839:T1)
            }
          }
        }
        frame #3 {
          n905 = case shown="True" w1840 {
            tunnel: [w1844 w1847] -> w1842
            tunnel: w1843 -> [_ w1846]
            tunnel: w1841 -> [w1844 w1845]
            frame False {
            }
            frame True {
              n906 = Build Array (concatenate)(w1845, w1846) -> (w1847:T1)
            }
          }
        }
      }
    }
    n907 = local read "Labels LSI336"() -> (w816:string[])
    n908 = Array Size(array=w816) -> (size(s)=w815:i32)
    n909 = local read "Plot selecter LSI336 \n     1      2     3     4"() -> (w824:bool[][])
    n910 = for {
      N: w815 -> [_]
      tunnel: w824 -> [w1705]
      shift-right: [w1699] -> w822
      shift-left: w823 -> [w1714]
      shift-right: [w1695] -> w821
      shift-left: w823 -> [w1712]
      shift-right: [w1696] -> w820
      shift-left: w823 -> [w1711]
      shift-right: [w1694] -> w819
      shift-left: w823 -> [w1710]
      tunnel: w784 -> [w1702]
      tunnel: w786 -> [w1700]
      i -> [w1703]
      n911 = Index Array(array=w1702, index (col)=w1703) -> (element=w1701:dbl[])  [unwired: 1 in]
      n912 = Index Array(array=w1705, index (row) #1=w1703, index (col) #1=0 ("index (row)"), index (row) #2=w1703, index (col) #2=1 ("index (row)"), index (row) #3=w1703, index (col) #3=2 ("index (row)"), index (row) #4=w1703, index (col) #4=3 ("index (row)")) -> (element #1=w1704:bool, element #2=w1698:bool, element #3=w1697:bool, element #4=w1693:bool)
      n913 = Bundle("TimeArray"=w1700, "DataArray"=w1701) -> (w1713:T26)  [unwired: 1 in]
      n914 = stacked-sequence {
        tunnel: w1714 -> [w1718 _ _ _]
        tunnel: [w1717 _ _ _] -> w1699
        tunnel: w1713 -> [w1716 w1726 w1734 w1742]
        tunnel: w1712 -> [_ w1725 _ _]
        tunnel: [_ w1724 _ _] -> w1695
        tunnel: [_ _ w1733 _] -> w1696
        tunnel: w1711 -> [_ _ w1732 _]
        tunnel: [_ _ _ w1741] -> w1694
        tunnel: w1710 -> [_ _ _ w1740]
        tunnel: w1704 -> [w1715 _ _ _]
        tunnel: w1698 -> [_ w1723 _ _]
        tunnel: w1697 -> [_ _ w1731 _]
        tunnel: w1693 -> [_ _ _ w1739]
        frame #0 {
          n915 = case shown="False" w1715 {
            tunnel: w1716 -> [_ w1720]
            tunnel: w1718 -> [w1719 w1722]
            tunnel: [w1719 w1721] -> w1717
            frame False {
            }
            frame True {
              n916 = Build Array (concatenate)(w1722, w1720) -> (w1721:T1)
            }
          }
        }
        frame #1 {
          n917 = case shown="True" w1723 {
            tunnel: [w1727 w1730] -> w1724
            tunnel: w1726 -> [_ w1728]
            tunnel: w1725 -> [w1727 w1729]
            frame False {
            }
            frame True {
              n918 = Build Array (concatenate)(w1729, w1728) -> (w1730:T1)
            }
          }
        }
        frame #2 {
          n919 = case shown="True" w1731 {
            tunnel: [w1735 w1738] -> w1733
            tunnel: w1734 -> [_ w1736]
            tunnel: w1732 -> [w1735 w1737]
            frame False {
            }
            frame True {
              n920 = Build Array (concatenate)(w1737, w1736) -> (w1738:T1)
            }
          }
        }
        frame #3 {
          n921 = case shown="True" w1739 {
            tunnel: [w1743 w1746] -> w1741
            tunnel: w1742 -> [_ w1744]
            tunnel: w1740 -> [w1743 w1745]
            frame False {
            }
            frame True {
              n922 = Build Array (concatenate)(w1745, w1744) -> (w1746:T1)
            }
          }
        }
      }
    }
    n923 = Array Size(array=w786) -> (size(s)=→"TimeArray Size (336)":i32)
    n924 = Array Size(array=w784) -> (size(s)=→"DataArray size (336)":i32[])
    n925 = Build Array (concatenate)(w836, w835, w820, w798) -> (→"Graph 3":T20)
    n926 = Build Array (concatenate)(w841, w842, w822, w800) -> (→"Graph 1":T20)
    n927 = Build Array (concatenate)(w839, w837, w821, w799) -> (→"Graph 2":T20)
    n928 = Build Array (concatenate)(w834, w833, w819, w797) -> (→"Graph 4":T20)
    n929 = Send Notification(notification="Stop Button", notifier=w758, error in (no error)=w757) -> (notifier out=w754:refnum<notifier>, error out=w755:errorcluster)
    "Cycle #" <- w767
  }
  n930 = while {
    shift-right: [w1941] -> _
    shift-left: refnum<class "DMMsData.lvclass"> refnum ("DMMsData in") -> [w1940]
    tunnel: errorcluster {"status"=FALSE, "code"=0, "source"=""} ("error in (no error)") -> [w1939]
    shift-right: [w1938] -> _
    shift-left: _ -> [_]
    tunnel: w3 -> [w1936]
    tunnel: w2 -> [w1935]
    tunnel: [w1934] -> w1
    i -> [w1937]
    stop <- w1933 stop-if-true
    n931 = Wait (ms)(milliseconds to wait="Measurement Interval DMMs (ms)") -> ()  [unwired: 1 out]
    n932 = Equal?(x=w1937, y=0) -> (x = y?=w1942:bool)
    n933 = case shown="True" "Measure DMMs?" {
      tunnel: w1942 -> [_ w1953]
      tunnel: [w1946 w1951] -> w1941
      tunnel: w1940 -> [w1946 w1950]
      tunnel: w1939 -> [w1945 w1949]
      tunnel: [w1945 w1948] -> w1938
      tunnel: w1937 -> [_ w1947]
      frame False {
      }
      frame True {
        n934 = Or(x="Initialize (DMMs)", y=w1953) -> (x .or. y?=w1952:bool)
        n935 = case shown="False" w1952 {
          tunnel: w1950 -> [w1968 w1985]
          tunnel: [w1965 w1984] -> w1951
          tunnel: w1949 -> [w1967 w1980]
          tunnel: [w1966 w1976] -> w1948
          tunnel: w1947 -> [w1964 _]
          frame False {
            n936 = local read "DMMsConfig"() -> (w1960:T10)
            n937 = call-dynamic "DMMs_measure.vi"("Sample #"="Sample #", "error in (no error)"=w1967, "MeasurementIndex"=w1964, "DMMsData in"=w1968) -> ("error out"=w1966:errorcluster, "DataArray"=w1958:dbl[][], "LastData"=→"DMM LastMeasurements":dbl[], "DMMsData out"=w1965:refnum<class "DMMsData.lvclass">, "DeviceActive?"=→"Active?":bool[], "TimeArray"=w1963:timestamp[])  [unwired: 2 in]
            n938 = Array Size(array=w1960) -> (size(s)=w1959:i32)
            n939 = for {
              N: w1959 -> [_]
              tunnel: w1963 -> [w1971]
              tunnel: w1958 -> [w1975]
              shift-right: [w1969] -> w1956
              shift-left: T1 [] -> [w1970]
              i -> [w1974]
              n940 = Index Array(array=w1975, index (col)=w1974) -> (element=w1973:dbl[])  [unwired: 1 in]
              n941 = Bundle("TimeArray"=w1971, "DataArray"=w1973) -> (w1972:T26)  [unwired: 1 in]
              n942 = Build Array (concatenate)(w1970, w1972) -> (w1969:T1)
            }
            "Graph DMMs 2" <- w1956
            "Graph DMMs 1" <- w1956
          }
          frame True {
            n943 = local write "Initialize (DMMs)"(FALSE ("Initialize 2")) -> ()
            n944 = local read "RUN Identifier"() -> (w1979:string)
            n945 = local read "Base Path"() -> (w1981:path)
            n946 = call-dynamic "DMMs_initialize.vi"("RunIdentifier"=w1979, "InstName"="InstName DMMs", "error in (no error)"=w1980, "base path"=w1981, "DMMsConfig"="DMMsConfig", "DMMsData in"=w1985) -> ("error out"=w1976:errorcluster, "DMMsLabels"=w1977:string[], "FileName"=→"DMMFileName":string, "DMMsData out"=w1984:refnum<class "DMMsData.lvclass">)  [unwired: 2 in]
            "DMMsLabels" <- w1977
            n947 = stacked-sequence {
              tunnel: w1977 -> [w1987 w2010]
              frame #0 {
                n948 = Array Size(array=w1987) -> (size(s)=w1996:i32)
                n949 = control-ref of="Graph DMMs 1"() -> (w1993:refnum<vi>)
                n950 = property class="XYGraph (strict)"(reference=w1993, error in=errorcluster {"status"=FALSE, "code"=0, "source"=""} ("error in (no error)")) -> (reference out=w1989:refnum<vi>, error out=w1992:errorcluster, "LegNumRows"=w1994:u32)
                n951 = for {
                  N: w1994 -> [_]
                  shift-right: [w2005] -> w1995
                  shift-left: w1992 -> [w2006]
                  tunnel: w1989 -> [w2004]
                  tunnel: [w2003] -> w1988 mode=indexing
                  i -> [w2008]
                  n952 = property class="XYGraph (strict)"(reference=w2004, error in=w2006, "Active Plot"=w2008, "Plot.Plot Name"="") -> (reference out=w2003:refnum<vi>, error out=w2005:errorcluster)
                }
                n953 = for {
                  N: w1996 -> [_]
                  shift-right: [w2000] -> w1990
                  shift-left: w1995 -> [w2001]
                  tunnel: w1988 -> [w1998] mode=indexing
                  tunnel: w1987 -> [w1997] mode=indexing
                  i -> [w2002]
                  n954 = property class="XYGraph (strict)"(reference=w1998, error in=w2001, "Active Plot"=w2002, "Plot.Plot Name"=w1997, "Plot.Visible?"=TRUE ("Plot.Visible")) -> (error out=w2000:errorcluster)  [unwired: 1 out]
                }
                "error out (DMM graphs)" <- w1990
              }
              frame #1 {
                n955 = Array Size(array=w2010) -> (size(s)=w2018:i32)
                n956 = control-ref of="Graph DMMs 2"() -> (w2013:refnum<vi>)
                n957 = property class="XYGraph (strict)"(reference=w2013, error in=errorcluster {"status"=FALSE, "code"=0, "source"=""} ("error in (no error)")) -> (reference out=w2012:refnum<vi>, error out=w2015:errorcluster, "LegNumRows"=w2016:u32)
                n958 = for {
                  N: w2016 -> [_]
                  shift-right: [w2027] -> w2017
                  shift-left: w2015 -> [w2028]
                  tunnel: w2012 -> [w2026]
                  tunnel: [w2025] -> w2011 mode=indexing
                  i -> [w2030]
                  n959 = property class="XYGraph (strict)"(reference=w2026, error in=w2028, "Active Plot"=w2030, "Plot.Plot Name"="") -> (reference out=w2025:refnum<vi>, error out=w2027:errorcluster)
                }
                n960 = for {
                  N: w2018 -> [_]
                  shift-right: [w2022] -> w2009
                  shift-left: w2017 -> [w2023]
                  tunnel: w2011 -> [w2020] mode=indexing
                  tunnel: w2010 -> [w2019] mode=indexing
                  i -> [w2024]
                  n961 = property class="XYGraph (strict)"(reference=w2020, error in=w2023, "Active Plot"=w2024, "Plot.Plot Name"=w2019, "Plot.Visible?"=TRUE ("Plot.Visible")) -> (error out=w2022:errorcluster)  [unwired: 1 out]
                }
                n962 = local write "error out (DMM graphs)"(w2009) -> ()
              }
            }
          }
        }
        "error out (DMMs)" <- w1948
      }
    }
    n963 = Get Notifier Status(notifier=w1936, error in (no error)=w1935) -> (current notification=w1933:bool, error out=w1934:errorcluster)  [unwired: 3 out]
    "cycle # (DMMs)" <- w1937
  }
  n964 = Merge Errors(w1, w5) -> (w6:errorcluster)
  n965 = Release Notifier(notifier=w4, error in (no error)=w6) -> (error out=→"error out (notifier)":errorcluster)  [unwired: 1 in, 2 out]
  n966 = call-dynamic "USBData_terminate.vi"("error in (no error)"=w35, "USBData in"=w36) -> ("error out"=w37:errorcluster)  [unwired: 8 in, 1 out]
  n967 = call-dynamic "LSI336Data_terminate.vi"("error in (no error)"=w25, "LSI336Data in"=w26) -> ("error out"=w24:errorcluster)  [unwired: 8 in, 1 out]
  n968 = call-dynamic "USBData_terminate.vi"("error in (no error)"=w18, "USBData in"=w19) -> ("error out"=w20:errorcluster)  [unwired: 8 in, 1 out]
  n969 = call "LSI218Data_terminate.vi"("error in (no error)"=w29, "LSI218Data in"=w30) -> ("error out"=w28:errorcluster)  [unwired: 8 in, 1 out]
  n970 = local write "error out (USB6210)"(w37) -> ()
  n971 = local write "error out (LSI336)"(w24) -> ()
  n972 = local write "error out (USB6210)"(w20) -> ()
  n973 = local write "error out (LSI218)"(w28) -> ()
